vi "SMain.vi"() -> ()   [LabVIEW 2011] (continued)
                            n859 = local read "测试项目及频点在txt输出"() -> (w1500:string)
                            n860 = Concatenate Strings(w1502, w1500) -> (w1501:string)
                          }
                          frame #11 {
                            w1544 = u16 3 items=["Normal Input", "Start", "Product Inf", "End"] ("Summary Method")
                            n861 = Or(x=w1539, y=w1538) -> (x .or. y?=w1537:bool)
                            n862 = local write "proBar"(u8 97 ("proBar")) -> ()
                            n863 = case shown="假" w1537 {
                              tunnel: w1545 -> [w1549 _]
                              tunnel: w1535 -> [w1548 _]
                              tunnel: w1536 -> [w1547 _]
                              tunnel: [w1546 "demo or manual mode" ("source")] -> w1504
                              frame False {
                                n864 = case shown="\"LX MCU\"" w1548 {
                                tunnel: w1549 -> [w1554 _ _]
                                tunnel: w1547 -> [_ w1558 w1562]
                                tunnel: [w1550 w1555 w1560] -> w1546
                                frame "NI PCI-6509", Default {
                                n865 = local read "Switch array"() -> (w1552:bool[][])
                                n866 = call "6509 simple.vi"("index (row)"=i8 79, "array input: P0-P1-P2-P3-P4-P5"=w1552, "DAQ device"=w1554) -> ("error out"=w1551:errorcluster)  [unwired: 4 in]
                                n867 = Unbundle By Name(w1551) -> ("source"=w1550:string)  [unwired: 2 out]
                                }
                                frame "LX MCU" {
                                w1557 = u16 1 items=["Testing", "Close All"] ("Function")
                                n868 = call "MCU Switch Control.vi"("Function"=w1557, "VISA"=w1558) -> ("error out"=w1556:errorcluster)  [unwired: 9 in]
                                n869 = Unbundle By Name(w1556) -> ("source"=w1555:string)  [unwired: 2 out]
                                }
                                frame "LX MCU_40G" {
                                w1561 = u16 1 items=["Testing", "Close All"] ("Function")
                                n870 = call "40G MCU Switch Control.vi"("Function"=w1561, "VISA"=w1562) -> ("error out"=w1559:errorcluster)  [unwired: 9 in]
                                n871 = Unbundle By Name(w1559) -> ("source"=w1560:string)  [unwired: 2 out]
                                }
                                }
                              }
                              frame True {
                              }
                            }
                            n872 = local read "Start Time"() -> (w1541:timestamp)
                            n873 = Get Date/Time In Seconds() -> (seconds since 1Jan1904=w1540:timestamp)
                            n874 = Subtract(x=w1540, y=w1541) -> (x-y=w1542:dbl)
                            n875 = Number To Fractional String(number=w1542) -> (F-format string=w1527:string)  [unwired: 3 in]
                            n876 = call "Summary Generating.vi"("Summary Method"=w1544, "Status String"=w1543, "Test Taking Time(s)"=w1527) -> ()  [unwired: 25 in]
                            n877 = Concatenate Strings("switch status:" ("字符串"), w1504) -> (w1523:string)
                            n878 = local read "SparaReult"() -> (w1521:bool)
                            n879 = local read "NEXTReult"() -> (w1520:bool)
                            n880 = local read "FEXTReult"() -> (w1519:bool)
                            n881 = local read "EEResult"() -> (w1511:bool)
                            n882 = Compound Arithmetic op=AND(w1521, w1520, w1519, w1511) -> (w1518:bool)
                            "test result" <- w1518
                            n883 = case shown="假" w1518 {
                              tunnel: [TRUE ("可见") TRUE ("可见")] -> w1517
                              tunnel: ["Testing Pass" ("文本.文本") "Testing Fail" ("文本.文本")] -> w1516
                              tunnel: [u32 6618880 u32 16711680] -> w1515
                              tunnel: [u32 40 ("文本.字体:字号") u32 40 ("文本.字体:字号")] -> w1514
                              frame True {
                              }
                              frame False {
                              }
                            }
                            n884 = property on="Result" class="Str"("Visible"=w1517, "Text.Text"=w1516, "Text.TextColor"=w1515, "Text.FontSize"=w1514, "DisabledEnum"=1, "Blinking"=FALSE ("闪烁")) -> ()  [unwired: 2 in, 2 out]
                            n885 = Format Date/Time String(time format string (%c)="%a %p %H:%M:%S %Y/%m/%d China Time.  Test Time: ") -> (date/time string=w1529:string)  [unwired: 2 in]
                            n886 = Format Date/Time String(time format string (%c)="%Y/%m/%d %H:%M:%S" ("时间格式字符串(%c)")) -> (date/time string=w1510:string)  [unwired: 2 in]
                            n887 = local read "test time"() -> (w1508:string[])
                            n888 = Concatenate Strings("Ended Test At " ("字符串"), w1529, w1527, "s" ("字符串"), "\n", w1523) -> (w1532:string)
                            n889 = call <vilib>:"Trim Whitespace.vi"("string"=w1510) -> ("trimmed string"=w1507:string)  [unwired: 1 in]
                            n890 = Concatenate Strings(w1526, "\r", w1532) -> (→"txt summary":string)
                            n891 = case shown="真" "Auto Count:" {
                              frame False {
                              }
                              frame True {
                                n892 = local read "Report No."() -> (w1576:string)
                                n893 = local read "Sample #"() -> (w1575:string)
                                n894 = local read "S/N:"() -> (w1577:string)
                                n895 = call "SN Report Number Increase.vi"("Sample #"=w1575, "Report No."=w1576, "S/N:"=w1577) -> ("Sample # out"=w1572:string, "Report No. out"=w1573:string, "S/N_out"=w1574:string)  [unwired: 6 in]
                                n896 = local write "S/N:"(w1574) -> ()
                                n897 = local write "Report No."(w1573) -> ()
                                n898 = local write "Sample #"(w1572) -> ()
                              }
                            }
                            n899 = Insert Into Array(array=w1508, new element=w1507) -> (w1506:string[])  [unwired: 1 in]
                            n900 = local write "test time"(w1506) -> ()
                          }
                          frame #12 {
                            n901 = local read "SparaReult"() -> (w1598:bool)
                            n902 = local read "NEXTReult"() -> (w1597:bool)
                            n903 = local read "FEXTReult"() -> (w1596:bool)
                            n904 = local read "EEResult"() -> (w1595:bool)
                            n905 = local read "SparaReults"() -> (w1587:bool[])
                            n906 = local read "NEXTReults"() -> (w1588:bool[])
                            n907 = property on="Test Status:" class="Str"() -> ("Value"=→"Test Status: 2":string)  [unwired: 2 in, 2 out]
                            n908 = Compound Arithmetic op=AND(w1598, w1597, w1596, w1595) -> (w1592:bool)
                            n909 = Insert Into Array(array=w1587, new element=w1588) -> (→"TestResult":bool[])  [unwired: 1 in]
                            n910 = local read "FullXml"() -> (w1580:bool)
                            n911 = local read "正常工单?"() -> (w1582:bool)
                            n912 = local read "打印模式"() -> (w1591:enum16{"IT Print", "EE Print"})
                            n913 = local read "测试模式"() -> (w1585:u16)
                            n914 = Equal?(x=w1585, y=u16 0) -> (x = y?=w1583:bool)
                            "测试模式" <- w1583
                            n915 = local read "EEUPLOAD"() -> (w1578:bool)
                            n916 = Equal?(x=w1591, y=enum16{"IT Print", "EE Print"}."IT Print") -> (x = y?=w1584:bool)
                            n917 = Compound Arithmetic op=AND(w1580, w1584, w1583, w1582) -> (w1579:bool)
                            n918 = Or(x=w1578, y=w1579) -> (x .or. y?=w1581:bool)
                            n919 = case shown="真" w1581 {
                              tunnel: w1593 -> [_ w1600]
                              tunnel: w1592 -> [_ w1599]
                              frame False {
                              }
                              frame True {
                                n920 = stacked-sequence {
                                seq-local: [w1616 _ _ _ _ _] -> [_ _ _ _ _ _]
                                seq-local: [w1615 _ _ _ _ _] -> [_ _ _ _ _ _]
                                tunnel: w1600 -> [_ _ _ _ _ _]
                                tunnel: w1599 -> [_ _ _ _ w1687 _]
                                frame #0 {
                                # "得到测试结果"
                                n921 = local read "条码输出"() -> (w1605:string)
                                n922 = property on="Current Testing Label/当前测试条码" class="Str"() -> ("Value"=w1614:string)  [unwired: 2 in, 2 out]
                                n923 = Equal?(x=w1605, y="nolabel") -> (x = y?=w1602:bool)
                                n924 = local read "Impedance Spec String"() -> (w1620:string)
                                n925 = String Length(string=w1605) -> (length=w1613:i32)
                                n926 = String Length(string=w1614) -> (length=w1612:i32)
                                n927 = local read "original Path"() -> (w1631:path)
                                n928 = local read "Diff Test Item Name"() -> (w1607:string[])
                                n929 = local read "TDR Test Item Name"() -> (w1606:string[])
                                n930 = call "_wmg_ImpSpecDivided@_XML.vi"("Input"=w1620, "input_dbl_stopTime"=2.0) -> ("OUTPUT2"=w1618:string[][], "Output"=w1619:string[][])
                                n931 = Greater?(x=w1612, y=w1613) -> (0:w1603:bool)
                                n932 = Or(x=w1603, y=w1602) -> (x .or. y?=w1601:bool)
                                n933 = Select(t=w1614, s=w1601, f=w1605) -> (s? t:f=→"usedSN":string)
                                n934 = Index Array(array=w1619, index (col) #1=0 ("禁用的索引 (列)"), index (col) #2=1 ("索引 (列)")) -> (element #1=w1647:string[], element #2=w1646:string[])  [unwired: 2 in]
                                n935 = Index Array(array=w1618, index (col)=1 ("禁用的索引 (列)")) -> (element=w1643:string[])  [unwired: 1 in]
                                n936 = Index Array(array=w1618, index (col)=3 ("禁用的索引 (列)")) -> (element=w1642:string[])  [unwired: 1 in]
                                n937 = Insert Into Array(array=w1607, new element=w1606) -> ()  [unwired: 1 in, 1 out]
                                n938 = call "readFromTXTForXMLFiles.vi"("input_path_dataSource"=w1631, "input_array_startTime"=w1647, "input_array_endTime"=w1646) -> ("show_Terminal Point"=w1616:dbl[], "show_array_TDD11"=→"show_TDD11":string[], "show_array_SDD21"=→"show_SDD21":string[], "show_array_SDD11_Max"=→"show_SDD11":string[], "show_array_ILD_Max"=→"show_ILD":string[], "show_array_SCC11_Max"=→"show_SCC11":string[], "show_array_Next"=→"show_Next":string[], "show_Cable Point"=w1615:dbl[], "show_array_TDD22"=→"show_TDD22":string[])  [unwired: 2 in, 2 out]
                                "show_Terminal Point" <- w1616
                                "show_Cable Point" <- w1615
                                n939 = Index Array(array=w1643, index #1=0 ("索引"), index #2=1 ("索引")) -> (element #1=w1635:string, element #2=w1632:string)
                                n940 = Index Array(array=w1642, index #1=0 ("索引"), index #2=1 ("索引")) -> (element #1=w1637:string, element #2=w1633:string)
                                n941 = local read "SparaReults"() -> (w1610:bool[])
                                n942 = local read "NEXTReults"() -> (w1609:bool[])
                                n943 = Insert Into Array(array=w1610, new element=w1609) -> (→"secondresult":bool[])  [unwired: 1 in]
                                n944 = Concatenate Strings(w1637, ":", w1635) -> (w1630:string)
                                n945 = Concatenate Strings(w1633, ":", w1632) -> (w1629:string)
                                n946 = Build Array(w1630, w1629) -> (→"show_impspec":string[])
                                }
                                frame #1 {
                                n947 = local read "TestResultSave"() -> (w1650:bool)
                                n948 = case shown="真" w1650 {
                                frame False {
                                }
                                frame True {
                                n949 = local read "auto get refer point"() -> (w1665:bool)
                                n950 = local read "width1"() -> (w1664:i32)
                                n951 = local read "width2"() -> (w1663:i32)
                                n952 = local read "show_TDD11"() -> (w1662:string[])
                                n953 = local read "show_TDD22"() -> (w1661:string[])
                                n954 = local read "test time"() -> (w1660:string[])
                                n955 = local read "show_impspec"() -> (w1659:string[])
                                n956 = local read "TestResult"() -> (w1651:bool[])
                                n957 = local read "FileName"() -> (w1658:string)
                                n958 = local read "FileVersion"() -> (w1657:string)
                                n959 = Bundle By Name(cluster="TestResultSummary", "auto get refer point"=w1665, "width1"=w1664, "width2"=w1663, "show_TDD11"=w1662, "show_TDD22"=w1661, "test time"=w1660, "show_impspec"=w1659, "TestResult"=w1651, "FileName"=w1658, "FileVersion"=w1657) -> (w1655:T9)
                                n960 = local read "original Path"() -> (w1654:path)
                                n961 = Build Path(base path=w1654, name or relative path="TXT\\TestResultSummary.txt" ("名称或相对路径")) -> (appended path=w1652:path)
                                n962 = call "TestResultSave.vi"("TestResultSummary"=w1655, "FileSavePath"=w1652) -> ()  [unwired: 10 in]
                                }
                                }
                                }
                                frame #2 {
                                n963 = local read "FileVersion"() -> (w1677:string)
                                n964 = local read "FileName"() -> (w1676:string)
                                n965 = local read "test time"() -> (w1681:string[])
                                n966 = local read "original Path"() -> (w1675:path)
                                n967 = local read "show_impspec"() -> (w1682:string[])
                                n968 = local read "usedSN"() -> (w1667:string)
                                n969 = local read "show_Terminal Point"() -> (w1680:dbl[])
                                n970 = local read "show_Cable Point"() -> (w1679:dbl[])
                                n971 = local read "sSpec"() -> (w1678:T3[])
                                n972 = local read "cluResult"() -> (w1674:T2)
                                n973 = Bundle By Name(cluster=T18 {"FileVersion"="DevelopmentSystem", "FileName"="DevelopmentSystem", "test time"=["2016/11/14 11:59:03"], "original Path"=path "D:/高频房软件/2. HPTS_VNA_Rev2.7.1.3-1107最新源码/Demo_data", "show_impspec"=[], "usedSN"="", "show_Terminal Point"=[], "show_Cable Point"=[], "sSpec"=[], "resultCluster"={"itemResult"=[], "itemName"=[]}, "customerPN"=""} ("xml_info"), "FileVersion"=w1677, "FileName"=w1676, "test time"=w1681, "original Path"=w1675, "show_impspec"=w1682, "usedSN"=w1667, "show_Terminal Point"=w1680, "show_Cable Point"=w1679, "sSpec"=w1678, "resultCluster"=w1674) -> (w1671:T18)
                                n974 = local read "TXT Data Path"() -> (w1673:path)
                                n975 = control-ref of="Test Status:"() -> (w1666:refnum<vi>)
                                n976 = local read "uploadPara"() -> (w1670:T1)
                                n977 = Build Path(base path=w1673, name or relative path="xml_info_new.txt") -> (appended path=w1668:path)
                                n978 = call "cluster_save.vi"("INI Fomatted Cluster"=w1671, "FileSavePath"=w1668) -> ()  [unwired: 9 in, 1 out]
                                n979 = local read "PN TYpe"() -> (w1669:string)
                                n980 = call "generateUploadZip.vi"("textRef"=w1666, "xmlPath"=w1668, "uploadPara"=w1670, "SN"=w1667, "pnType"=w1669) -> ()  [unwired: 14 in, 1 out]
                                }
                                frame #3 {
                                n981 = First Call?() -> (First Call?: T/F=w1684:bool)
                                n982 = case shown="真" w1684 {
                                frame False {
                                }
                                frame True {
                                (unwired) "net use \\\\172.20.20.86 Luxshare-ict /user:C040345" ("standard input")
                                n983 = local read "NetCmd"() -> (w1685:string)
                                n984 = call <vilib>:"System Exec.vi"("command line"=w1685) -> ()  [unwired: 7 in, 4 out]
                                }
                                }
                                }
                                frame #4 {
                                n985 = local read "CountXmlPath"() -> (w1688:path)
                                n986 = local read "usedSN"() -> (w1686:string)
                                n987 = call "xmlNodecreate.vi"("SN"=w1686, "TestResult"=w1687, "path"=w1688) -> ()  [unwired: 1 in, 1 out]
                                }
                                frame #5 {
                                n988 = local read "CountXmlPath"() -> (w1693:path)
                                n989 = call "xmlConfigRead.vi"("path to XML document"=w1693, "XPath expression"="//FailedSN/*") -> ("OutParaArray"=w1695:string[])  [unwired: 2 out]
                                n990 = call "xmlConfigRead.vi"("path to XML document"=w1693, "XPath expression"="//PassedSN/*") -> ("OutParaArray"=w1696:string[])  [unwired: 2 out]
                                n991 = Array Size(array=w1696) -> (size(s)=w1692:i32)
                                n992 = Array Size(array=w1695) -> (size(s)=w1691:i32)
                                n993 = Add(x=w1691, y=w1692) -> (x+y=w1690:i32)
                                n994 = Equal To 0?(x=w1690) -> (x = 0?=w1694:bool)
                                n995 = case shown="假" w1694 {
                                tunnel: w1691 -> [w1703 _]
                                tunnel: w1690 -> [w1701 _]
                                tunnel: [w1702 0.0] -> w1689
                                frame False {
                                n996 = Divide(x=w1703, y=w1701) -> (x/y=w1699:dbl)
                                n997 = Multiply(x=w1699, y=100) -> (x*y=w1702:dbl)
                                }
                                frame True {
                                }
                                }
                                n998 = local write "Passed"(w1692) -> ()
                                n999 = local write "Failed"(w1691) -> ()
                                n1000 = local write "Total"(w1690) -> ()
                                n1001 = local write "ratio"(w1689) -> ()
                                }
                                }
                              }
                            }
                          }
                          frame #13 {
                            n1002 = property on="Tester:" class="Ring (严格)"() -> ("RingText.Text"=w1723:string)  [unwired: 2 in, 2 out]
                            n1003 = property on="Approval:" class="Ring (严格)"() -> ("RingText.Text"=w1722:string)  [unwired: 2 in, 2 out]
                            n1004 = local read "PN Des"() -> (w1727:string)
                            n1005 = local read "P/N:"() -> (w1726:string)
                            n1006 = Format Date/Time String(time format string (%c)="%Y-%m-%d") -> (date/time string=w1721:string)  [unwired: 2 in]
                            n1007 = Build Array("Applicant:", w1727, w1726, "Report No.", "Sample #", w1723, w1722, w1721) -> (w1717:string[])
                            n1008 = local read "Items Result"() -> (w1716:string[])
                            n1009 = local read "EEResult"() -> (w1711:bool)
                            n1010 = local read "FEXT Result"() -> (w1713:string[])
                            n1011 = local read "NEXT Result"() -> (w1714:string[])
                            n1012 = local read "NEXT?"() -> (w1719:bool)
                            n1013 = local read "FEXT?"() -> (w1718:bool)
                            n1014 = local read "Thru?"() -> (w1720:bool)
                            n1015 = stacked-sequence {
                              frame #0 {
                                w1741 = ";" ("字符串")
                                n1016 = local read "Reference"() -> (w1747:T5)
                                n1017 = local read "SparaReult"() -> (w1734:bool)
                                n1018 = local read "NEXTReult"() -> (w1733:bool)
                                n1019 = local read "FEXTReult"() -> (w1732:bool)
                                n1020 = local read "EEResult"() -> (w1731:bool)
                                n1021 = Unbundle(w1747) -> ("db_ResultString"=w1746:refnum<vi>)  [unwired: 3 out]
                                n1022 = property class="Str"(reference=w1746) -> ("Value"=w1739:string)  [unwired: 1 in, 2 out]
                                n1023 = Compound Arithmetic op=AND(w1734, w1733, w1732, w1731) -> (w1730:bool)
                                n1024 = local read "db_VNA"() -> (w1745:string)
                                n1025 = Search and Replace String(replace all?=TRUE ("替换全部？(F)"), input string=w1739, search string="\n", replace string="," ("替换字符串(\"\")")) -> (result string=w1735:string)  [unwired: 4 in, 3 out]
                                n1026 = Select(t="PASS", s=w1730, f="FAIL") -> (s? t:f=w1742:string)
                                n1027 = Concatenate Strings(w1745, w1735, w1741, w1742, w1741) -> (w1740:string)
                                n1028 = local write "db_VNA"(w1740) -> ()
                              }
                              frame #1 {
                                w1749 = ";" ("字符串")
                                n1029 = local read "Applicant:"() -> (w1752:string)
                                n1030 = local read "db_VNA"() -> (w1753:string)
                                n1031 = property on="Tester:" class="Ring (严格)"() -> ("RingText.Text"=w1751:string)  [unwired: 2 in, 2 out]
                                n1032 = property on="Approval:" class="Ring (严格)"() -> ("RingText.Text"=w1750:string)  [unwired: 2 in, 2 out]
                                n1033 = Concatenate Strings(w1753, w1752, w1749, w1751, w1749, w1750, w1749) -> (w1748:string)
                                n1034 = local write "db_VNA"(w1748) -> ()
                              }
                              frame #2 {
                                w1758 = ";" ("字符串")
                                n1035 = local read "start"() -> (w1761:timestamp)
                                n1036 = Get Date/Time In Seconds() -> (seconds since 1Jan1904=w1760:timestamp)
                                n1037 = Subtract(x=w1760, y=w1761) -> (x-y=w1762:dbl)
                                n1038 = Number To Fractional String(number=w1762, precision (6)=i16 2 ("精度(6)")) -> (F-format string=w1756:string)  [unwired: 2 in]
                                n1039 = local read "db_VNA"() -> (w1767:string)
                                n1040 = String To IP() -> (0:w1764:u32)  [unwired: 1 in]
                                n1041 = Format Date/Time String(time format string (%c)="%H:%M:%S %Y/%m/%d") -> (date/time string=w1766:string)  [unwired: 2 in]
                                n1042 = IP To String(2:w1764) -> (0:w1763:string)  [unwired: 1 in]
                                n1043 = Concatenate Strings(w1756, "S" ("字符串")) -> (w1754:string)
                                n1044 = Concatenate Strings(w1767, w1766, w1758, w1754, w1758, w1763, w1758, "EEPROM:OK", w1758) -> (w1765:string)
                                n1045 = local write "db_VNA"(w1765) -> ()
                              }
                            }
                            n1046 = Build Array(w1720, w1719, w1718, w1711) -> (w1712:bool[])
                            n1047 = Build Array(w1716, w1714, w1713) -> (w1715:string[][])
                            n1048 = for {
                              tunnel: w1712 -> [w1772] mode=indexing
                              shift-right: [w1770] -> w1708
                              shift-left: w1717 -> [w1771]
                              tunnel: w1715 -> [w1769] mode=indexing
                              n1049 = case shown="真" w1772 {
                                tunnel: w1771 -> [w1773 w1778]
                                tunnel: [w1773 w1777] -> w1770
                                tunnel: w1769 -> [_ w1776]
                                frame False {
                                }
                                frame True {
                                n1050 = Array To Spreadsheet String(array=w1776, 3:"%s" ("格式字符串")) -> (spreadsheet string=w1775:string)  [unwired: 1 in]
                                n1051 = call <vilib>:"Trim Whitespace.vi"("string"=w1775) -> ("trimmed string"=w1774:string)  [unwired: 1 in]
                                n1052 = Insert Into Array(array=w1778, new element=w1774) -> (w1777:string[])  [unwired: 1 in]
                                }
                              }
                            }
                            "Report Inf" <- w1708
                            n1053 = local read "original Path"() -> (w1710:path)
                            n1054 = Array To Spreadsheet String(array=w1708, 3:"%s" ("格式字符串")) -> (spreadsheet string=w1707:string)  [unwired: 1 in]
                            n1055 = Build Path(base path=w1710, name or relative path="TXT\\ReportInf.txt" ("名称或相对路径")) -> (appended path=w1706:path)
                            n1056 = Write to Text File(file (use dialog)=w1706, text=w1707) -> ()  [unwired: 2 in, 3 out]
                          }
                          frame #14 {
                            # "生成报告"
                            n1057 = property on="MO:" class="Str"() -> ("Visible"=w1782:bool)  [unwired: 2 in, 2 out]
                            n1058 = case shown="真" w1782 {
                              tunnel: w1789 -> [_ w1814]
                              frame False {
                              }
                              frame True {
                                w1794 = "0"
                                w1795 = "1"
                                n1059 = property class="Str"(reference=w1814) -> (reference out=w1807:refnum<vi>, "Value"=w1808:string)  [unwired: 1 in, 1 out]
                                n1060 = local read "DB1"() -> (w1790:T8)
                                n1061 = local read "test result"() -> (w1805:bool)
                                n1062 = local read "MO:"() -> (w1812:string)
                                n1063 = local read "P/N:"() -> (w1813:string)
                                n1064 = call "按工单数量查询.vi"("MO"=w1812, "DBSet"=w1790, "test result"=w1805, "PN"=w1813) -> ("当前数量"=w1804:string)  [unwired: 5 in]
                                n1065 = Decimal String To Number(string=w1804) -> (number=w1803:i32)  [unwired: 2 in, 1 out]
                                n1066 = local write "Pro Num"(w1803) -> ()
                                n1067 = Concatenate Strings(w1808, "\n", "当前工单已生产：" ("字符串"), w1804, "条" ("字符串")) -> (w1806:string)
                                n1068 = local read "MO Num"() -> (w1801:i64)
                                n1069 = local read "Pro Num"() -> (w1802:i64)
                                n1070 = property class="Str"(reference=w1807, "Value"=w1806) -> ()  [unwired: 1 in, 2 out]
                                n1071 = Subtract(x=w1802, y=w1801) -> (x-y=w1799:i64)
                                n1072 = Greater?(x=w1799, y=i64 0) -> (0:w1797:bool)
                                n1073 = Greater?(x=w1799, y=i64 20) -> (0:w1796:bool)
                                n1074 = Select(t=w1795, s=w1797, f=w1794) -> (s? t:f=w1793:string)
                                n1075 = Select(t=w1795, s=w1796, f=w1794) -> (s? t:f=w1792:string)
                                n1076 = Concatenate Strings(w1793, w1792) -> (w1791:string)
                                n1077 = case shown="\"10\"" w1791 {
                                frame "00", Default {
                                w1815 = u32 0
                                n1078 = property on="Pro Num" class="DigNum (严格)"("NumText.TextColor"=w1815) -> ()  [unwired: 2 in, 2 out]
                                n1079 = property on="P/N:" class="Str"("Text.TextColor"=w1815) -> ()  [unwired: 2 in, 2 out]
                                }
                                frame "10" {
                                w1816 = u32 16772608
                                n1080 = property on="Pro Num" class="DigNum (严格)"("NumText.TextColor"=w1816) -> ()  [unwired: 2 in, 2 out]
                                n1081 = property on="P/N:" class="Str"("Text.TextColor"=w1816) -> ()  [unwired: 2 in, 2 out]
                                }
                                frame "11" {
                                w1817 = u32 14423296
                                n1082 = property on="Pro Num" class="DigNum (严格)"("NumText.TextColor"=w1817) -> ()  [unwired: 2 in, 2 out]
                                n1083 = property on="P/N:" class="Str"("Text.TextColor"=w1817) -> ()  [unwired: 2 in, 2 out]
                                }
                                }
                              }
                            }
                            n1084 = local read "Report Temp. Name"() -> (w1787:string)
                            n1085 = local read "TXT Data Path"() -> (w1781:path)
                            n1086 = local read "Report Config"() -> (w1786:string[])
                            n1087 = local read "Report Inf"() -> (w1785:string[])
                            n1088 = local read "Excel?"() -> (w1788:bool)
                            n1089 = Strip Path(path=w1781) -> (stripped path=w1780:path)  [unwired: 1 out]
                            n1090 = case shown="真" w1788 {
                              tunnel: w1781 -> [_ w1819]
                              tunnel: w1787 -> [_ w1830]
                              tunnel: w1786 -> [_ w1831]
                              tunnel: w1785 -> [_ w1826]
                              tunnel: w1784 -> [_ w1820]
                              tunnel: w1780 -> [_ w1818]
                              frame False {
                              }
                              frame True {
                                n1091 = Index Array(array=w1831, index #1=0 ("索引")) -> (element #1=w1827:string, element #2=w1825:string)  [unwired: 1 in]
                                n1092 = String To Path(string=w1830) -> (path=w1829:path)
                                n1093 = call "Excel Config.vi"("Config String"=w1827) -> ("Start(0,0)"=w1834:cluster{i32, i32}[], "Sheet Number List"=w1833:i32[], "File Name List"=w1832:string[])  [unwired: 8 in]
                                n1094 = call "Excel Config.vi"("Config String"=w1825) -> ("Start(0,0)"=w1824:cluster{i32, i32}[])  [unwired: 8 in, 2 out]
                                n1095 = call "Excel Export.vi"("template Path"=w1829, "Data Basic Path"=w1819, "File Name List"=w1832, "Sheet Index List"=w1833, "Report Inf"=w1826, "Inf start"=w1824, "Sheet start(0,0)"=w1834, "Demo"=w1820, "Report Type"="Report Type:", "reportSavePath"=w1818, "StartPage"="Start Page", "EndPage"="End Page") -> ()  [unwired: 15 in, 1 out]
                              }
                            }
                            n1096 = local write "proBar"(u8 90 ("proBar")) -> ()
                          }
                          frame #15 {
                            (unwired) FALSE
                            # "上传测试数据"
                            n1097 = local read "EEPROMTF"() -> (w1839:bool)
                            n1098 = local read "upload"() -> (w1838:bool)
                            n1099 = local read "测试模式"() -> (w1837:bool)
                            n1100 = Or(x=w1838, y=w1839) -> (x .or. y?=w1836:bool)
                            n1101 = And(x=w1836, y=w1837) -> (x .and. y?=w1835:bool)
                            n1102 = case shown="真" w1835 {
                              tunnel: w1840 -> [_ w1842]
                              frame False {
                                n1103 = local write "proBar"(u8 99 ("proBar")) -> ()
                              }
                              frame True {
                                n1104 = case shown="假" w1842 {
                                frame True {
                                n1105 = local read "strFSN 原始SN"() -> (w1847:string)
                                n1106 = local read "NetPathCompress1"() -> (w1845:path)
                                n1107 = local read "NetCmdCompress"() -> (w1846:string)
                                n1108 = local read "NetPathCompress2"() -> (w1844:path)
                                n1109 = call <vilib>:"Application Directory.vi"() -> ("Application Directory"=w1850:path)
                                n1110 = Build Path(base path=w1850, name or relative path="Demo_data") -> (appended path=w1848:path)
                                n1111 = local read "EEPROMTF"() -> (w1855:bool)
                                n1112 = local read "db_VNA"() -> (w1853:string)
                                n1113 = local read "条码输出"() -> (w1851:string)
                                n1114 = local read "Excel?"() -> (w1854:bool)
                                n1115 = local read "P/N:"() -> (w1856:string)
                                n1116 = local read "S/N:"() -> (w1852:string)
                                n1117 = call "compressFiles-Demo.vi"("mis原始sn字符串"=w1847, "P/N:"=w1856, "NetPathCompress1"=w1845, "NetPathCompress2"=w1844, "NetCmdCompress"=w1846, "original Path"=w1848, "EEPROMTF"=w1855, "Excel?"=w1854, "db_VNA"=w1853, "S/N:"=w1852, "条码输出"=w1851) -> ()  [unwired: 5 in]
                                }
                                frame False {
                                n1118 = local read "重测原因"() -> (w1859:string)
                                n1119 = property on="测试模式" class="Ring (严格)"() -> ("RingText.Text"=w1858:string)  [unwired: 2 in, 2 out]
                                n1120 = property on="线别" class="Ring (严格)"() -> ("RingText.Text"=w1857:string)  [unwired: 2 in, 2 out]
                                n1121 = local read "MO:"() -> (w1860:string)
                                n1122 = local read "Current Testing Label/当前测试条码"() -> (w1871:string)
                                n1123 = local read "要烧录的时间和Sn"() -> (w1864:string)
                                n1124 = local read "NetCmdCompress"() -> (w1861:string)
                                n1125 = local read "NetPathCompress1"() -> (w1862:path)
                                n1126 = local read "customer date"() -> (w1870:string)
                                n1127 = local read "strFSN 原始SN"() -> (w1873:string)
                                n1128 = local read "NetPathCompress2"() -> (w1863:path)
                                n1129 = local read "未经进制转换的sn(客户 jin zhi sn)"() -> (w1865:string)
                                n1130 = local read "Shi jin zhi sn"() -> (w1869:string)
                                n1131 = local read "midVar_time_date"() -> (w1868:timestamp)
                                n1132 = Format Date/Time String(time format string (%c)="%Y%m%d" ("时间格式字符串(%c)"), seconds (now)=w1868) -> (date/time string=w1866:string)  [unwired: 1 in]
                                n1133 = local read "original Path"() -> (w1874:path)
                                n1134 = local read "EEPROMTF"() -> (w1879:bool)
                                n1135 = local read "db_VNA"() -> (w1877:string)
                                n1136 = local read "条码输出"() -> (w1875:string)
                                n1137 = local read "Excel?"() -> (w1878:bool)
                                n1138 = local read "P/N:"() -> (w1880:string)
                                n1139 = local read "S/N:"() -> (w1876:string)
                                n1140 = local read "要烧录的DateCode"() -> (w1872:string)
                                n1141 = call "compressFiles.vi"("original Path"=w1874, "重测原因"=w1859, "NetPathCompress2"=w1863, "EEPROMTF"=w1879, "Excel?"=w1878, "测试模式"=w1858, "db_VNA"=w1877, "P/N:"=w1880, "S/N:"=w1876, "测试线别"=w1857, "NetPathCompress1"=w1862, "NetCmdCompress"=w1861, "mis原始sn字符串"=w1873, "条码输出"=w1875, "eprm_datecode"=w1872, "eprm_dateAndsn"=w1864, "itsn_really"=w1871, "label_date"=w1870, "decimel_sn"=w1869, "label_sn"=w1865, "decimel_date"=w1866, "MO"=w1860) -> ()  [unwired: 6 in]
                                }
                                }
                                n1142 = local write "proBar"(u8 95 ("proBar")) -> ()
                              }
                            }
                          }
                          frame #16 {
                            n1143 = flat-sequence {
                              frame #0 {
                                n1144 = local read "AutoSN"() -> (w1881:bool)
                                n1145 = call "运行批处理.vi"() -> ()  [unwired: 12 in]
                                n1146 = local write "proBar"(u8 100 ("proBar")) -> ()
                                n1147 = case shown="假" w1881 {
                                frame False {
                                n1148 = local write "S/N:"("" ("S/N:")) -> ()
                                n1149 = property on="S/N:" class="Str"("DisabledEnum"=T17."Enabled" ("禁用")) -> ()  [unwired: 2 in, 2 out]
                                }
                                frame True {
                                n1150 = local write "S/N:"("automatic sn" ("S/N:")) -> ()
                                n1151 = property on="S/N:" class="Str"("DisabledEnum"=T17."Disabled and Grayed Out" ("禁用")) -> ()  [unwired: 2 in, 2 out]
                                }
                                }
                                n1152 = disable-structure shown="启用" {
                                frame Disabled {
                                n1153 = call <vilib>:"System Exec.vi"("run minimized? (F)"=TRUE, "command line"="taskkill /IM bartend.exe /F") -> ()  [unwired: 6 in, 4 out]
                                }
                                frame Enabled {
                                }
                                }
                              }
                              frame #1 {
                                w1889 = FALSE ("Urgent Stop")
                                w1893 = 0
                                n1154 = property on="Start Test" class="Bool"("DisabledEnum"=w1893) -> ()  [unwired: 2 in, 2 out]
                                n1155 = property on="Tab_Graph" class="TabCtl (严格)"("Value"=w1893) -> ()  [unwired: 2 in, 2 out]
                                n1156 = property on="Urgent Stop" class="Bool (严格)"("DisabledEnum"=2 ("索引")) -> ()  [unwired: 2 in, 2 out]
                                n1157 = local write "State"("wait" ("state")) -> ()
                                n1158 = local write "Urgent Stop"(w1889) -> ()
                                n1159 = global write "全局.vi" "manual stop"(w1889) -> ()
                                n1160 = property on="S/N:" class="Str"("Key Focus"=TRUE ("键选中")) -> ()  [unwired: 2 in, 2 out]
                              }
                            }
                          }
                        }
                      }
                    }
                  }
                }
              }
              frame #3 {
                n1161 = local read "caliFlag"() -> (w1894:string)
                n1162 = case shown="\"假\", 默认" w1894 {
                  frame "假", Default {
                  }
                  frame "cali" {
                    n1163 = local write "State"("datacheck" ("state")) -> ()
                    n1164 = property on="Start Test" class="Bool"("DisabledEnum"=T17."Disabled and Grayed Out" ("禁用")) -> ()  [unwired: 2 in, 2 out]
                    n1165 = property on="Tab_Graph" class="TabCtl (严格)"("Value"=T15."Sxxxx1" ("Tab_Graph")) -> ()  [unwired: 2 in, 2 out]
                  }
                }
              }
            }
          }
          frame "datacheck" {
            n1166 = stacked-sequence {
              frame #0 {
                n1167 = local read "original Path"() -> (w1903:path)
                n1168 = Build Path(base path=w1903, name or relative path="txt" ("名称或相对路径")) -> (appended path=w1898:path)
                n1169 = call "caliCalcu.vi"("basic"=w1898) -> ("FileExsit"=w1901:bool, "keyValue"=w1900:string[][])  [unwired: 9 in]
                n1170 = case shown="真" w1901 {
                  tunnel: w1900 -> [_ w1912]
                  tunnel: [_ w1913] -> w1899
                  frame False {
                  }
                  frame True {
                    n1171 = local read "sampleData"() -> (w1919:string)
                    n1172 = Spreadsheet String To Array(format string="%f" ("格式字符串"), spreadsheet string=w1919, array type (2D Dbl)=dbl[][] []) -> (array=w1918:dbl[][])  [unwired: 1 in]
                    n1173 = Fract/Exp String To Number(string=w1912) -> (number=w1916:dbl[][])  [unwired: 3 in, 1 out]
                    n1174 = Subtract(x=w1916, y=w1918) -> (x-y=w1909:dbl[][])
                    n1175 = Array To Spreadsheet String(array=w1912, 3:"%f" ("格式字符串")) -> (spreadsheet string=→"caliData":string)  [unwired: 1 in]
                    n1176 = Absolute Value(x=w1916) -> (abs(x)=w1907:dbl[][])
                    n1177 = Absolute Value(x=w1909) -> (abs(x)=w1908:dbl[][])
                    n1178 = Divide(x=w1908, y=w1907) -> (x/y=w1915:dbl[][])
                    n1179 = Less Or Equal?(x=w1915, y=0.1) -> (x <= y?=w1905:bool[][])
                    n1180 = Not A Number/Path/Refnum?(number/path/refnum=w1907) -> (NaN/Path/Refnum?=w1906:bool[][])
                    n1181 = Or(x=w1906, y=w1905) -> (x .or. y?=w1904:bool[][])
                    n1182 = And Array Elements(Boolean array=w1904) -> (logical AND=w1913:bool)
                  }
                }
                "caliPassed" <- w1899
              }
              frame #1 {
                n1183 = local read "caliPassed"() -> (w1921:bool)
                n1184 = case shown="假" w1921 {
                  frame False {
                    n1185 = One Button Dialog(message="校准数据超出10%范围，未通过" ("消息")) -> ()  [unwired: 1 in, 1 out]
                  }
                  frame True {
                    n1186 = local read "caliData"() -> (w1923:string)
                    n1187 = local read "SystemMode"() -> (w1928:string)
                    n1188 = Format Date/Time String() -> (date/time string=w1927:string)  [unwired: 3 in]
                    n1189 = property on="sampleNo" class="Ring (严格)"() -> ("RingText.Text"=w1932:string)  [unwired: 2 in, 2 out]
                    n1190 = property on="Type" class="Ring (严格)"() -> ("RingText.Text"=w1931:string)  [unwired: 2 in, 2 out]
                    n1191 = Build Array(w1932, w1931, "Figo", "PASS", w1928, w1923, w1927) -> (w1926:string[])
                    n1192 = for {
                      shift-right: [w1937] -> w1925
                      shift-left: "INSERT INTO dbo.cali_log (goldenSampleNo, type, caliUser, result, setNo, detail, caliDate)\nVALUES ('@goldensampleno', '@type', '@caliuser', '@result', '@setno', '@detail', '@calidate')" -> [w1938]
                      tunnel: string[] ["@goldensampleno", "@type", "@caliuser", "@result", "@setno", "@detail", "@calidate"] -> [w1936] mode=indexing
                      tunnel: w1926 -> [w1935] mode=indexing
                      n1193 = Search and Replace String(input string=w1938, search string=w1936, replace string=w1935) -> (result string=w1937:string)  [unwired: 5 in, 3 out]
                    }
                    n1194 = local read "DB1"() -> (w1924:T8)
                    n1195 = call "query.net.vi"("Sql"=w1925, "DBSet"=w1924) -> ()  [unwired: 8 in, 2 out]
                  }
                }
              }
              frame #2 {
                n1196 = local read "caliPassed"() -> (w1939:bool)
                n1197 = case shown="真" w1939 {
                  frame False {
                  }
                  frame True {
                    n1198 = One Button Dialog(message="校准通过，可以开始测试" ("消息")) -> ()  [unwired: 1 in, 1 out]
                  }
                }
              }
              frame #3 {
                n1199 = local write "State"("wait" ("State")) -> ()
              }
              frame #4 {
                n1200 = local read "P/N:"() -> (w1942:string)
                n1201 = property on="P/N:" class="Str"("Val(Sgnl)"=w1942) -> ()  [unwired: 2 in, 2 out]
              }
            }
          }
          frame "exit" {
          }
          frame "wait", Default {
            n1202 = event shown="[8] \"Manual\": 值改变" {
              selector: _ -> [_ _ _ _ _ _ _ _ _ _ _ _ _ _ _ _ _ _ _ _]
              dyn-events: _ -> [_ _ _ _ _ _ _ _ _ _ _ _ _ _ _ _ _ _ _ _]
              timeout: _ -> [_ _ _ _ _ _ _ _ _ _ _ _ _ _ _ _ _ _ _ _]
              tunnel: ["Stop" _ _ w1996 _ _ _ _ _ _ _ _ _ _ _ _ _ _ _ _] -> w1944
              event "Stop": Value Change {
                n1203 = event-data() -> ()  [unwired: 1 in, 5 out]
              }
              event "save config": Value Change {
                n1204 = event-data() -> ()  [unwired: 1 in, 5 out]
                n1205 = case shown="真" "save config" {
                  frame False {
                  }
                  frame True {
                    n1206 = stacked-sequence {
                      seq-local: [w1953 _ _] -> [_ w1984 _]
                      frame #0 {
                        n1207 = local read "Crosstalk  by Trace"() -> (w1964:bool)
                        n1208 = local read "Local Database"() -> (w1967:bool)
                        n1209 = local read "By Channel?"() -> (w1952:bool)
                        n1210 = local read "Use Counts?"() -> (w1949:bool)
                        n1211 = property on="VNA Model:" class="Enum (严格)"() -> ("RingText.Text"=w1971:string)  [unwired: 2 in, 2 out]
                        n1212 = property on="DAQ  Model:" class="Enum (严格)"() -> ("RingText.Text"=w1970:string)  [unwired: 2 in, 2 out]
                        n1213 = property on="DAQ Device" class="Ring (严格)"() -> ("RingText.Text"=w1969:string)  [unwired: 2 in, 2 out]
                        n1214 = local read "Dem 2X"() -> (w1963:bool)
                        n1215 = local read "Manual"() -> (w1965:bool)
                        n1216 = property on="VNA VISA" class="VISAName"() -> ("Text.Text"=w1972:string)  [unwired: 2 in, 2 out]